vi "SMain.vi"() -> ()   [LabVIEW 2011] (continued)
      n242 = call "deleteFolder_vna.vi"("input_path"=w507) -> ()  [unwired: 1 in]
      n243 = Build Path(base path=w495, name or relative path="DelayConfig.txt" ("名称或相对路径")) -> (appended path=w493:path)
      n244 = call <vilib>:"Check if File or Folder Exists.vi"("path"=w493) -> ("file or folder exists?"=w492:bool, "dup path"=w491:path)  [unwired: 8 in, 1 out]
      n245 = call <vilib>:"Application Directory.vi"() -> ("Application Directory"=w516:path)
      n246 = constructor class="CPLTSApplicationClass"() -> (reference out=w504:refnum<k24>)  [unwired: 3 in, 2 out]
      n247 = call "equipconfirm.vi"("path to XML document"=w458) -> ("确认结果"=w457:bool)
      n248 = Build Path(base path=w516, name or relative path="Database\\LabelList.xlsx" ("名称或相对路径")) -> (appended path=w514:path)
      n249 = call <vilib>:"Check if File or Folder Exists.vi"("path"=w514) -> ("error out"=w511:errorcluster, "file or folder exists?"=w513:bool, "dup path"=w512:path)  [unwired: 8 in]
      n250 = local read "打印模式"() -> (w503:enum16{"IT Print", "EE Print"})
      n251 = case shown="假" w457 {
        frame False {
          n252 = Quit LabVIEW(quit? (T)=TRUE ("退出？(T)")) -> ()
        }
        frame True {
        }
      }
      n253 = control-ref of="Test Status:"() -> (w414:refnum<vi>)
      n254 = case shown="真" w492 {
        tunnel: w491 -> [w553 w564]
        frame False {
          w549 = 100.0 ("写入延时（单位：ms）")
          w550 = 100.0 ("读取延时（单位：ms）")
          n255 = local write "读取延时（单位：ms）"(w550) -> ()
          n256 = global write "延时设置全局变量.vi" "写入延时"(w550) -> ()
          n257 = local write "Q写入延时（单位：ms）"(250.0 ("写入延时（单位：ms）")) -> ()
          n258 = local write "S写入延时（单位：ms）"(w549) -> ()
          n259 = global write "延时设置全局变量.vi" "写入延时"(w549) -> ()
          n260 = call-poly <vilib>:"Write To Spreadsheet File.vi"("2D data"=string[][] [["Q写入延时时间（ms）：", "250"], ["S写入延时时间（ms）：", "100"], ["读取延时时间（ms）：", "100"]], "file path (dialog if empty)"=w553) -> ()  [unwired: 6 in, 1 out]
        }
        frame True {
          n261 = call-poly <vilib>:"Read From Spreadsheet File.vi"("file path (dialog if empty)"=w564) -> ("all rows"=w563:string[][])  [unwired: 6 in, 4 out]
          n262 = Index Array(array=w563, index (col)=1 ("禁用的索引 (列)")) -> (element=w561:string[])  [unwired: 1 in]
          n263 = Index Array(array=w561, index #1=0 ("索引")) -> (element #1=w559:string, element #2=w557:string, element #3=w556:string)  [unwired: 2 in]
          n264 = Fract/Exp String To Number(string=w559) -> (number=w554:dbl)  [unwired: 3 in, 1 out]
          n265 = Fract/Exp String To Number(string=w556) -> (number=w558:dbl)  [unwired: 3 in, 1 out]
          n266 = Fract/Exp String To Number(string=w557) -> (number=w555:dbl)  [unwired: 3 in, 1 out]
          n267 = local write "Q写入延时（单位：ms）"(w554) -> ()
          n268 = global write "延时设置全局变量.vi" "写入延时"(w554) -> ()
          n269 = local write "S写入延时（单位：ms）"(w555) -> ()
          n270 = local write "读取延时（单位：ms）"(w558) -> ()
          n271 = global write "延时设置全局变量.vi" "读取延时"(w558) -> ()
        }
      }
      n272 = invoke class="CPLTSApplicationClass" method="ShowWindow"(reference=w504, "nCmdShow"="nCmdShow") -> (reference out=w506:refnum<k24>)  [unwired: 2 in, 3 out]
      n273 = case shown="\"IT Print\", 默认" w503 {
        frame "IT Print", Default {
          n274 = property on="MO:" class="Str"("Visible"=TRUE ("可见")) -> ()  [unwired: 2 in, 2 out]
        }
        frame "EE Print" {
          n275 = property on="MO:" class="Str"("Visible"=FALSE ("可见")) -> ()  [unwired: 2 in, 2 out]
        }
      }
      n276 = property on="属性节点" class="Str"(reference=w414, "Text.BGColor"=u32 16711680, "Text.TextColor"=u32 16448250) -> ()  [unwired: 1 in, 2 out]
      n277 = case shown="真" w482 {
        tunnel: w458 -> [_ w526]
        tunnel: [string[] ["net use \\\\172.200.20.86 Luxshare-ict /user:C040345", "\\\\172.20.20.86\\HuaweiData\\DataRoot\\XML", "net use \\\\172.20.20.113 mesuser /user:mesuser", "\\\\172.20.20.113\\emc\\HPTS\\VNA", "\\\\172.20.20.113\\emc\\HPTS\\SI", "false"] ("OutParaArray") w535] -> w481
        tunnel: [string[] ["false"] ("OutParaArray") w533] -> w464
        tunnel: ["A" ("node text") w529] -> w459
        tunnel: [string[] [] ("OutParaArray") w527] -> w443
        frame False {
        }
        frame True {
          w539 = "Mo" ("名称")
          w541 = "PN" ("名称")
          n278 = call "xmlConfigRead.vi"("path to XML document"=w526, "XPath expression"="//OtherPara/*") -> ("OutParaArray"=w533:string[])  [unwired: 2 out]
          n279 = call "xmlConfigRead.vi"("path to XML document"=w526, "XPath expression"="//UploadPara/*") -> ("OutParaArray"=w535:string[])  [unwired: 2 out]
          n280 = call "xmlConfigRead.vi"("path to XML document"=w526, "XPath expression"="//LastPartNo/*") -> ("OutParaVariant"=w543:variant)  [unwired: 2 out]
          n281 = call "xmlConfigRead.vi"("path to XML document"=w526, "XPath expression"="//LineID/Line/@Name") -> ("OutParaArray"=w524:string[])  [unwired: 2 out]
          n282 = call "xmlConfigRead.vi"("path to XML document"=w526, "XPath expression"="//DBSet/ConnectInfo/@*") -> ("OutParaArray"=w527:string[])  [unwired: 2 out]
          n283 = call "xmlConfigRead.vi"("path to XML document"=w526, "XPath expression"="//SystemList/CurrentNO/@Name") -> ("OutParaArray"=w531:string[])  [unwired: 2 out]
          n284 = Get Variant Attribute(Variant=w543, name=w541) -> (duplicate Variant=w544:variant, value=w542:variant)  [unwired: 2 in, 2 out]
          n285 = Get Variant Attribute(Variant=w544, name=w539) -> (value=w540:variant)  [unwired: 2 in, 3 out]
          n286 = property on="线别" class="Ring (严格)"("Strings []"=w524) -> ()  [unwired: 2 in, 2 out]
          n287 = Variant To Data(type=w539, Variant=w540) -> (data=w537:string)  [unwired: 1 in, 1 out]
          n288 = Variant To Data(type=w541, Variant=w542) -> (data=w538:string)  [unwired: 1 in, 1 out]
          n289 = property on="P/N:" class="Str"("Val(Sgnl)"=w538) -> ()  [unwired: 2 in, 2 out]
          n290 = local write "MO:"(w537) -> ()
          n291 = Index Array(array=w531, index=0 ("索引")) -> (element=w529:string)
        }
      }
      "SystemMode" <- w459
      n292 = case shown="假" w513 {
        tunnel: w512 -> [w576 _]
        tunnel: w511 -> [_ _]
        frame False {
          n293 = call <vilib>:"New Report.vi"("report type"=T16."Excel") -> ("report out"=w578:refnum<class "NI_report.lvclass">)  [unwired: 13 in, 1 out]
          n294 = call <vilib>:"Excel Get Worksheet.vi"("report in"=w578, "worksheet index (0)"=0) -> ("report out"=w580:refnum<class "NI_report.lvclass">, "error out"=w579:errorcluster)  [unwired: 12 in]
          n295 = Build Array(string[] ["料号", "日期类型", "年份起始位", "年份结束位", "周起始位", "周结束位", "月份起始位", "月份结束位", "天数起始位", "天数结束位", "流水号起始位", "流水号起始位"]) -> (w573:string[][])
          n296 = call-poly <vilib>:"Excel Easy Table.vi"("report in"=w580, "text data"=w573, "error in (no error)"=w579) -> ("report out"=w575:refnum<class "NI_report.lvclass">)  [unwired: 8 in, 4 out]
          n297 = call-dynamic "Save Report to File.vi"("report in"=w575, "report file path"=w576) -> ("report out"=w583:refnum<class "NI_report.lvclass">, "error out"=w582:errorcluster)  [unwired: 12 in]
          n298 = call-dynamic "Dispose Report.vi"("report in"=w583, "wait until printing completed? (T)"=TRUE, "error in (no error)"=w582) -> ()  [unwired: 12 in, 1 out]
        }
        frame True {
        }
      }
      n299 = local write "Excel?"(TRUE ("Excel?")) -> ()
      n300 = local write "upload"(TRUE ("upload")) -> ()
      n301 = invoke class="CPLTSApplicationClass" method="CloseAllFiles"(reference=w506) -> ()  [unwired: 2 in, 3 out]
      n302 = constructor class="LabelPrintHelper"() -> (reference out=→"PRINT":refnum<k24>)  [unwired: 3 in, 2 out]
      n303 = constructor class="MESDataServices"() -> (reference out=→"SN":refnum<k24>)  [unwired: 3 in, 2 out]
      n304 = Delete From Array(array=w443, length=4 ("长度")) -> (deleted portion=w434:string[], array with subset deleted=w442:string[])  [unwired: 1 in]
      n305 = Index Array(array=w442) -> (element #1=w441:string, element #2=w440:string, element #3=w438:string, element #4=w439:string)  [unwired: 4 in]
      n306 = global write "全局.vi" "print templete"(FALSE ("print templete")) -> ()
      n307 = call "DES.vi"("sourceData"=w438, "操作"=enum16{"DES_Encrypt", "DES_Decrypt"}."DES_Decrypt") -> ("加密后字符串"=w437:string)  [unwired: 8 in, 1 out]
      n308 = Index Array(array=w464, index #1=0 ("索引"), index #2=1 ("索引"), index #3=2 ("索引"), index #4=3 ("索引")) -> (element #1=w461:string, element #2=w454:string, element #3=w450:string, element #4=w445:string)
      n309 = Decimal String To Number(string=w445) -> (number=→"startSN":i32)  [unwired: 2 in, 1 out]
      n310 = Bundle By Name(cluster=w433, "Server"=w441, "DB"=w440, "PSW"=w437, "User"=w439) -> (→"DB1":T8)
      n311 = Decimal String To Number(string=w454) -> (number=w453:i32)  [unwired: 2 in, 1 out]
      n312 = Equal?(x=w461, y="true") -> (x = y?=→"ConvertStyle":bool)
      n313 = Index Array(array=w481, index #1=0 ("索引"), index #2=1 ("索引"), index #3=2 ("索引"), index #4=3 ("索引"), index #5=4 ("索引"), index #6=5 ("索引"), index #7=6 ("索引"), index #8=7 ("索引"), index #9=8 ("索引")) -> (element #1=→"NetCmd":string, element #2=→"NetPathHW":string, element #3=→"NetCmdCompress":string, element #4=w473:string, element #5=w472:string, element #6=w468:string, element #7=w420:string, element #8=→"NetTemppath":string, element #9=→"NetLocalpath":string)
      n314 = String To Path(string=w473) -> (path=→"NetPathCompress1":path)
      n315 = String To Path(string=w472) -> (path=→"NetPathCompress2":path)
      n316 = Equal?(x=w450, y="true") -> (x = y?=→"TestResultSave":bool)
      n317 = global write "全局.vi" "logsetting"(w453) -> ()
      n318 = Equal?(x=w468, y="true") -> (x = y?=→"AlarmDisplay":bool)
      n319 = Index Array(array=w434) -> (element #1=w432:string, element #2=w431:string, element #3=w429:string, element #4=w427:string)  [unwired: 4 in]
      n320 = call "DES.vi"("sourceData"=w429, "操作"=enum16{"DES_Encrypt", "DES_Decrypt"}."DES_Decrypt") -> ("加密后字符串"=w430:string)  [unwired: 8 in, 1 out]
      n321 = Equal?(x=w420, y="true") -> (x = y?=→"asychronus":bool)
      n322 = Bundle By Name(cluster=w433, "Server"=w432, "DB"=w431, "PSW"=w430, "User"=w427) -> (→"DB2":T8)
    }
    frame #5 {
      n323 = property on="Type" class="Ring (严格)"("Val(Sgnl)"=u16 0 ("值(信号)")) -> ()  [unwired: 2 in, 2 out]
      n324 = property on="Start Test" class="Bool"("BoolText.Text"="START TEST" ("布尔文本.文本")) -> ()  [unwired: 2 in, 2 out]
      n325 = local write "caliDataSelect"(FALSE ("caliDataSelect")) -> ()
    }
    frame #6 {
      n326 = while {
        tunnel: [w590] -> _
        stop <- w590 stop-if-true
        n327 = case shown="\"test\"" "State" {
          tunnel: [_ _ TRUE ("Stop") w1944] -> w590
          frame "test" {
            n328 = stacked-sequence {
              frame #0 {
                n329 = property on="Start Test" class="Bool"("DisabledEnum"=2) -> ()  [unwired: 2 in, 2 out]
                n330 = local write "proBar"(u8 0 ("proBar")) -> ()
                n331 = local write "preStation"("" ("preStation")) -> ()
                n332 = property on="preStation" class="Str"("Visible"=FALSE ("可见")) -> ()  [unwired: 2 in, 2 out]
                n333 = control-ref of="Test Status:"() -> (w592:refnum<vi>)
                n334 = property on="属性节点" class="Str"(reference=w592, "Text.BGColor"=u32 16448250, "Text.TextColor"=u32 0) -> ()  [unwired: 1 in, 2 out]
                n335 = property on="S/N:" class="Str"("DisabledEnum"=T17."Disabled and Grayed Out" ("禁用")) -> ()  [unwired: 2 in, 2 out]
                n336 = local write "strFSN 原始SN"("" ("strFSN 原始SN")) -> ()
                n337 = local write "Current Testing Label/当前测试条码"("") -> ()
                n338 = local write "midVar_time_date"(timestamp(3534465477 s since 1904-01-01) ("midVar_time_date")) -> ()
                n339 = local write "未经进制转换的sn(客户 jin zhi sn)"("" ("未经进制转换的sn(客户 jin zhi sn)")) -> ()
                n340 = local write "Test Status:"("" ("Test Status:")) -> ()
                n341 = local write "要烧录的DateCode"("" ("要烧录的DateCode")) -> ()
                n342 = local write "要烧录的时间和Sn"("" ("要烧录的时间和Sn")) -> ()
                "customer date" <- "" ("customer date")
                "Shi jin zhi sn" <- "" ("Shi jin zhi sn")
              }
              frame #1 {
                n343 = local read "Use Counts?"() -> (w610:bool)
                n344 = case shown="真" w610 {
                  tunnel: [TRUE w613] -> w609
                  frame False {
                  }
                  frame True {
                    n345 = stacked-sequence {
                      seq-local: [w616 _] -> [_ w624]
                      seq-local: [w615 _] -> [_ w621]
                      tunnel: [_ w620] -> w613
                      frame #0 {
                        n346 = local read "RS232 I2C Counts"() -> (w614:refnum<visa-resource-name>)
                        n347 = call "读取使用次数和寿命.vi"("截取长度"=4, "开始截取位"=8, "VISA  2"=w614) -> ("result"=w616:bool, "Data Out"=w615:u8[], "无符号字节数组"=→"无符号字节数组":u8[])  [unwired: 6 in]
                        "Data Out  2" <- w615
                        "result" <- w616
                      }
                      frame #1 {
                        # "读取使用次数错误吗？"
                        n348 = Equal?(x=FALSE, y=w624) -> (x = y?=w622:bool)
                        n349 = case shown="假" w622 {
                          tunnel: w621 -> [w643 _]
                          tunnel: [w636 FALSE] -> w620
                          frame False {
                            w630 = 256
                            # "使用次数大于寿命"
                            n350 = Index Array(array=w643, index #1=0 ("索引"), index #2=1 ("索引"), index #3=2 ("索引"), index #4=3 ("索引")) -> (element #1=w635:u8, element #2=w639:u8, element #3=w633:u8, element #4=w638:u8)
                            n351 = Multiply(x=w630, y=w635) -> (x*y=w634:i32)
                            n352 = Multiply(x=w630, y=w633) -> (x*y=w632:i32)
                            n353 = Add(x=w632, y=w638) -> (x+y=w629:i32)
                            n354 = Add(x=w634, y=w639) -> (x+y=w628:i32)
                            n355 = Subtract(x=w629, y=w628) -> (x-y=w627:i32)
                            n356 = Less?(x=w627, y=200) -> (x < y?=w625:bool)
                            n357 = case shown="真" w625 {
                              frame False {
                              }
                              frame True {
                                n358 = One Button Dialog(message="计数板可使用次数小于200,请注意！" ("消息")) -> ()  [unwired: 1 in, 1 out]
                              }
                            }
                            n359 = Greater?(x=w628, y=w629) -> (0:w637:bool)
                            n360 = case shown="假" w637 {
                              tunnel: [w646 FALSE] -> w636
                              frame False {
                                n361 = local read "RS232 I2C Counts"() -> (w645:refnum<visa-resource-name>)
                                n362 = call "使用次数加1.vi"("VISA  2"=w645) -> ("result"=w646:bool)  [unwired: 10 in]
                              }
                              frame True {
                              }
                            }
                            n363 = local write "UseAge"(w629) -> ()
                            n364 = local write "Used"(w628) -> ()
                          }
                          frame True {
                            n365 = One Button Dialog(message="测试板使用次数读取错误！") -> ()  [unwired: 1 in, 1 out]
                          }
                        }
                      }
                    }
                  }
                }
                n366 = local write "test time"(string[] [] ("test time")) -> ()
                n367 = case shown="真" w609 {
                  frame False {
                    # "测试版使用次数是否合格"
                    n368 = local read "UseAge"() -> (w654:i64)
                    n369 = local read "Used"() -> (w657:i64)
                    n370 = local write "Go"(FALSE ("Go")) -> ()
                    n371 = Number To Decimal String(number=w657) -> (decimal integer string=w656:string)  [unwired: 1 in]
                    n372 = Number To Decimal String(number=w654) -> (decimal integer string=w653:string)  [unwired: 1 in]
                    n373 = Concatenate Strings("测试板使用了", w656, "次,超过了最大使用寿命:" ("字符串"), w653, "不允许继续使用，请更换测试板后继续测试！" ("字符串"), "或者修改使用次数的动作失败！" ("字符串")) -> (w651:string)
                    n374 = One Button Dialog(message=w651) -> ()  [unwired: 1 in, 1 out]
                  }
                  frame True {
                    # "测试版使用次数是否合格"
                    n375 = local read "线别确认"() -> (w661:bool)
                    n376 = Not(x=w661) -> (.not. x?=w660:bool)
                    n377 = case shown="假" w660 {
                      frame False {
                        n378 = control-ref of="Test Status:"() -> (w667:refnum<vi>)
                        n379 = property class="Str"(reference=w667) -> (reference out=w665:refnum<vi>, "Value"=w668:string)  [unwired: 1 in, 1 out]
                        n380 = local read "DateCode8Value_0X30"() -> (w662:i32)
                        n381 = local read "打印模式"() -> (w671:enum16{"IT Print", "EE Print"})
                        n382 = local read "AutoSN"() -> (w672:bool)
                        n383 = local read "ConvertStyle"() -> (w670:bool)
                        n384 = Number To Hexadecimal String(2:w662) -> (0:w663:string)  [unwired: 1 in]
                        n385 = Concatenate Strings(w668, "\n", "当前datacode为:0X", w663) -> (w666:string)
                        n386 = property class="Str"(reference=w665, "Value"=w666) -> ()  [unwired: 1 in, 2 out]
                        n387 = case shown="假" w672 {
                          tunnel: w671 -> [_ w729]
                          tunnel: w670 -> [w682 w728]
                          tunnel: w662 -> [w681 w727]
                          frame False {
                            # "前站数据是否需要管控"
                            n388 = local read "S/N:"() -> (w679:string)
                            n389 = local read "P/N:"() -> (w674:string)
                            n390 = local read "DB1"() -> (w678:T8)
                            n391 = call "前站查询(T1).vi"("Station"="preStation", "Pre Check"="Pre Check", "PN"=w674, "DBSet"=w678, "SN"=w679) -> ("判定"=w677:bool)  [unwired: 6 in]
                            n392 = call "前站查询.vi"("DBSet"=w678, "SN"=w679) -> ("判定"=w676:bool)  [unwired: 9 in]
                            n393 = And(x=w676, y=w677) -> (x .and. y?=w675:bool)
                            n394 = case shown="真" w675 {
                              tunnel: w682 -> [_ w686]
                              tunnel: w681 -> [_ w685]
                              frame False {
                                n395 = One Button Dialog(message="前面有不良维修记录待处理，请进行处理后再测试" ("消息")) -> ()  [unwired: 1 in, 1 out]
                                n396 = local write "Go"(FALSE ("Go")) -> ()
                              }
                              frame True {
                                n397 = stacked-sequence {
                                tunnel: w686 -> [_ w694]
                                tunnel: w685 -> [_ w693]
                                frame #0 {
                                n398 = local read "DB1"() -> (w687:T8)
                                n399 = local read "LastSN"() -> (w691:string)
                                n400 = local read "S/N:"() -> (w690:string)
                                n401 = call "重测.vi"("Last SN"=w691, "DBSet"=w687, "SN"=w690) -> ("继续?"=→"继续?":bool, "重测原因"=→"重测原因":string)  [unwired: 6 in, 1 out]
                                }
                                frame #1 {
                                n402 = local read "继续?"() -> (w692:bool)
                                n403 = case shown="真" w692 {
                                tunnel: w694 -> [_ w706]
                                tunnel: w693 -> [_ w705]
                                frame False {
                                n404 = local write "Go"(FALSE ("Go")) -> ()
                                }
                                frame True {
                                # "20160919增加从labelprint表查询，理由：作业流程变更，第一站就打条码。"
                                # "针对重工已经打印标签\n的进行修改，从资讯\n数据库中查到SN对应\n的信息回来进行测试"
                                n405 = local read "DB1"() -> (w703:T8)
                                n406 = local read "P/N:"() -> (w725:string)
                                n407 = local read "Local Database"() -> (w697:bool)
                                n408 = local read "mid_str_labelType"() -> (w723:string)
                                n409 = local read "labelConfig"() -> (w722:string[])
                                n410 = local read "打印模式"() -> (w700:enum16{"IT Print", "EE Print"})
                                n411 = local read "校验信息"() -> (w702:T7)
                                n412 = Equal?(x=w700, y=enum16{"IT Print", "EE Print"}."EE Print") -> (x = y?=w698:bool)
                                n413 = Or(x=w697, y=w698) -> (x .or. y?=w696:bool)
                                n414 = local read "S/N:"() -> (w724:string)
                                "LastSN" <- w724
                                n415 = local read "mid_array_eep"() -> (w721:string[][])
                                n416 = call "精简框图4.vi"("P/N:"=w725, "mid_str_labelType"=w723, "DateCode8Value_0X30"=w705, "Convert Style"=w706, "LocalDataBase?"=w696, "labelConfig"=w722, "mid_array_eep"=w721, "SNKeep"="SN Keep", "S/N"=w724, "DBSet"=w703, "校验信息"=w702) -> ("show_date"=w710:timestamp, "要烧录的时间和Sn"=w720:string, "未经进制转换的sn(客户 jin zhi sn)"=w711:string, "要烧录的DateCode"=w719:string, "strFSN 原始 Customer sn"=w712:string, "输出的label内容"=w709:string, "Go"=w708:bool, "mid_array_temp_int"=w718:u8[][], "S/N:"=w717:string, "Customer Date"=w716:string, "shi jin zhi sn"=w715:string, "Report No."=w714:string, "Sample #"=w713:string)  [unwired: 4 in]
                                n417 = And(x=w708, y=TRUE) -> (x .and. y?=w707:bool)
                                n418 = local write "Go"(w707) -> ()
                                n419 = local write "midVar_time_date"(w710) -> ()
                                n420 = local write "strFSN 原始SN"(w712) -> ()
                                n421 = local write "未经进制转换的sn(客户 jin zhi sn)"(w711) -> ()
                                n422 = local write "要烧录的时间和Sn"(w720) -> ()
                                n423 = local write "要烧录的DateCode"(w719) -> ()
                                n424 = local write "Current Testing Label/当前测试条码"(w709) -> ()
                                n425 = local write "mid_array_temp_int"(w718) -> ()
                                n426 = local write "S/N:"(w717) -> ()
                                n427 = local write "customer date"(w716) -> ()
                                n428 = local write "Shi jin zhi sn"(w715) -> ()
                                n429 = local write "Report No."(w714) -> ()
                                n430 = local write "Sample #"(w713) -> ()
                                n431 = local write "midVar_str_SN"(w709) -> ()
                                }
                                }
                                }
                                }
                              }
                            }
                          }
                          frame True {
                            n432 = local write "重测原因"("firsttest" ("重测原因")) -> ()
                            n433 = case shown="\"IT Print\", 默认" w729 {
                              tunnel: w728 -> [w733 w762]
                              tunnel: w727 -> [w731 w756]
                              frame "IT Print", Default {
                                # "没有转进制的流水"
                                # "mid_array_temp_int 是展开后的烧录文件"
                                # "通过MIS获得Sn"
                                n434 = local read "MO:"() -> (w742:string)
                                n435 = local read "mid_str_labelType"() -> (w750:string)
                                n436 = local read "SN"() -> (w732:refnum<k24>)
                                n437 = local read "labelConfig"() -> (w749:string[])
                                n438 = local read "mid_array_eep"() -> (w748:string[][])
                                n439 = local read "P/N:"() -> (w751:string)
                                n440 = local read "校验信息"() -> (w730:T7)
                                n441 = call "精简框图3.vi"("P/N:"=w751, "mid_str_labelType"=w750, "DateCode8Value_0X30"=w731, "Convert Style"=w733, "新引用"=w732, "labelConfig"=w749, "mid_array_eep"=w748, "工单号"=w742, "校验信息"=w730) -> ("show_date"=w741:timestamp, "要烧录的时间和Sn"=→"要烧录的时间和Sn":string, "未经进制转换的sn(客户 jin zhi sn)"=w734:string, "要烧录的DateCode"=→"要烧录的DateCode":string, "strFSN 原始 Customer sn"=w737:string, "输出的label内容"=w740:string, "Go"=w743:bool, "mid_array_temp_int"=w747:u8[][], "S/N:"=w746:string, "Customer Date"=w736:string, "shi jin zhi sn"=w735:string, "Report No."=w745:string, "Sample #"=w744:string)  [unwired: 6 in]
                                "Current Testing Label/当前测试条码" <- w740
                                n442 = local write "mid_array_temp_int"(w747) -> ()
                                n443 = local write "S/N:"(w746) -> ()
                                n444 = local write "Report No."(w745) -> ()
                                n445 = local write "Sample #"(w744) -> ()
                                n446 = local write "midVar_str_SN"(w740) -> ()
                                n447 = local write "Go"(w743) -> ()
                                n448 = local write "midVar_time_date"(w741) -> ()
                                n449 = local write "未经进制转换的sn(客户 jin zhi sn)"(w734) -> ()
                                n450 = local write "strFSN 原始SN"(w737) -> ()
                                n451 = local write "customer date"(w736) -> ()
                                n452 = local write "Shi jin zhi sn"(w735) -> ()
                              }
                              frame "EE Print" {
                                n453 = local read "startSN"() -> (w753:i32)
                                n454 = control-ref of="Test Status:"() -> (w760:refnum<vi>)
                                n455 = local read "mid_str_labelType"() -> (w766:string)
                                n456 = local read "mid_str_snformat"() -> (w765:string)
                                n457 = local read "P/N:"() -> (w763:string)
                                n458 = local read "mid_array_eep"() -> (w761:string[][])
                                n459 = local read "校验信息"() -> (w752:T7)
                                n460 = property class="Str"(reference=w760) -> (reference out=w758:refnum<vi>, "Value"=w759:string)  [unwired: 1 in, 1 out]
                                n461 = call "精简框图1.vi"("mid_str_labelType"=w766, "mid_array_eep"=w761, "mid_str_snformat"=w765, "Convert Style"=w762, "DateCode8Value_0X30"=w756, "P/N"=w763, "Sart SN"=w753, "校验信息"=w752) -> ("LocalSN Generate Status"=w755:string, "midVar_time_date"=w767:timestamp, "midVar_str_SN"=w768:string, "mid_array_temp_int"=w769:u8[][], "S/N:"=w770:string, "Report No."=w771:string, "Sample #"=w772:string)  [unwired: 5 in]
                                n462 = Concatenate Strings(w759, "\n", w755) -> (w757:string)
                                n463 = local write "Go"(TRUE ("Go")) -> ()
                                n464 = local write "midVar_time_date"(w767) -> ()
                                n465 = local write "midVar_str_SN"(w768) -> ()
                                n466 = local write "mid_array_temp_int"(w769) -> ()
                                n467 = local write "S/N:"(w770) -> ()
                                n468 = local write "Report No."(w771) -> ()
                                n469 = local write "Sample #"(w772) -> ()
                                n470 = property class="Str"(reference=w758, "Value"=w757) -> ()  [unwired: 1 in, 2 out]
                              }
                            }
                          }
                        }
                      }
                      frame True {
                        n471 = disable-structure shown="禁用" {
                          frame Disabled {
                            # "前站数据是否需要管控"
                            n472 = local read "S/N:"() -> (w777:string)
                            n473 = call "subVI3_MAIN_checkBeforeTest_wmg.vi"("input_str_SN"=w777) -> ("show_bool_checkResult"=w776:bool, "show_str_failTable"=w778:string, "show_messageOut"=w775:string)  [unwired: 1 out]
                            n474 = case shown="真" w776 {
                              tunnel: w778 -> [w783 _]
                              tunnel: w775 -> [_ w788]
                              frame False {
                                w782 = "\n"
                                n475 = local write "Go"(FALSE ("Go")) -> ()
                                n476 = Concatenate Strings("工站", w782, w783, w782, "没有测试或者测试失败！") -> (w780:string)
                                n477 = One Button Dialog(message=w780) -> ()  [unwired: 1 in, 1 out]
                                n478 = local write "Test Status:"(w780) -> ()
                              }
                              frame True {
                                # "前站数据的查询结果"
                                n479 = local write "preStation"(w788) -> ()
                                n480 = local read "AutoSN"() -> (w786:bool)
                                n481 = property on="preStation" class="Str"("Visible"=TRUE ("可见")) -> ()  [unwired: 2 in, 2 out]
                                n482 = case shown="假" w786 {
                                frame False {
                                n483 = local read "mid_str_labelType"() -> (w792:string)
                                n484 = local read "mid_str_snformat"() -> (w791:string)
                                n485 = local read "mid_array_eep"() -> (w793:string[][])
                                n486 = local read "S/N:"() -> (w789:string)
                                n487 = local read "P/N:"() -> (w790:string)
                                n488 = call "精简框图2.vi"("S/N:"=w789, "P/N:"=w790, "mid_str_snformat"=w791, "mid_str_labelType"=w792, "mid_array_eep"=w793) -> ("Report No."=w794:string, "Sample #"=w795:string, "midVar_time_date"=w796:timestamp, "midVar_str_SN"=w797:string, "mid_array_temp_int"=w798:u8[][])  [unwired: 6 in]
                                n489 = local write "Report No."(w794) -> ()
                                n490 = local write "Sample #"(w795) -> ()
                                n491 = local write "midVar_time_date"(w796) -> ()
                                n492 = local write "midVar_str_SN"(w797) -> ()
                                n493 = local write "mid_array_temp_int"(w798) -> ()
                                }
                                frame True {
                                # "自动EE获取sn"
                                n494 = local read "mid_str_labelType"() -> (w801:string)
                                n495 = local read "mid_str_snformat"() -> (w800:string)
                                n496 = local read "mid_array_eep"() -> (w799:string[][])
                                n497 = call "精简框图1.vi"("mid_str_labelType"=w801, "mid_array_eep"=w799, "mid_str_snformat"=w800) -> ("midVar_time_date"=w802:timestamp, "midVar_str_SN"=w803:string, "mid_array_temp_int"=w804:u8[][], "S/N:"=w805:string, "Report No."=w806:string, "Sample #"=w807:string)  [unwired: 10 in, 1 out]
                                n498 = local write "midVar_time_date"(w802) -> ()
                                n499 = local write "midVar_str_SN"(w803) -> ()
                                n500 = local write "mid_array_temp_int"(w804) -> ()
                                n501 = local write "S/N:"(w805) -> ()
                                n502 = local write "Report No."(w806) -> ()
                                n503 = local write "Sample #"(w807) -> ()
                                }
                                }
                                n504 = local write "Go"(TRUE ("Go")) -> ()
                              }
                            }
                          }
                          frame Enabled {
                          }
                        }
                        n505 = local write "Go"(FALSE ("Go")) -> ()
                        n506 = One Button Dialog(message="线别未确认" ("消息")) -> ()  [unwired: 1 in, 1 out]
                      }
                    }
                  }
                }
              }
              frame #2 {
                n507 = local read "Go"() -> (w808:bool)
                n508 = case shown="真" w808 {
                  frame False {
                    w812 = 0
                    n509 = property on="S/N:" class="Str"("Key Focus"=TRUE ("键选中")) -> ()  [unwired: 2 in, 2 out]
                    n510 = local write "State"("wait" ("state")) -> ()
                    n511 = local write "S/N:"("") -> ()
                    n512 = property on="S/N:" class="Str"("DisabledEnum"=T17."Enabled" ("禁用")) -> ()  [unwired: 2 in, 2 out]
                    n513 = property on="Start Test" class="Bool"("DisabledEnum"=w812) -> ()  [unwired: 2 in, 2 out]
                    n514 = property on="Tab_Graph" class="TabCtl (严格)"("Value"=w812) -> ()  [unwired: 2 in, 2 out]
                  }
                  frame True {
                    n515 = local read "P/N:"() -> (w818:string)
                    n516 = local read "VNA Model:"() -> (w824:enum16{"E5071C", "N5230A(C)", "N5224A"})
                    n517 = local read "Spec _Col"() -> (w819:i32[])
                    n518 = control-ref of="Test Status:"() -> (w823:refnum<vi>)
                    n519 = local read "VNA VISA"() -> (w825:refnum<visa-resource-name>)
                    n520 = local read "S/N:"() -> (w822:string)
                    n521 = call "Sample name judge.vi"("Sample  Name:"=w818, "START input"=TRUE) -> ("START output"=w826:bool)
                    n522 = case shown="真" w826 {
                      tunnel: "DAQ Device" -> [_ w846]
                      tunnel: w825 -> [_ w845]
                      tunnel: w824 -> [_ w844]
                      tunnel: w823 -> [_ w843]
                      tunnel: w822 -> [_ w842]
                      tunnel: "Port Type" -> [_ w841]
                      tunnel: "Demo" -> [_ w840]
                      tunnel: w819 -> [_ w839]
                      tunnel: w818 -> [_ w838]
                      tunnel: "Manual" -> [_ w837]
                      tunnel: "VISA COM" -> [_ w836]
                      tunnel: "DAQ  Model:" -> [_ w835]
                      tunnel: "Crosstalk  by Trace" -> [_ w834]
                      frame False {
                        w833 = 0
                        n523 = property on="S/N:" class="Str"("Key Focus"=TRUE ("键选中")) -> ()  [unwired: 2 in, 2 out]
                        n524 = local write "State"("wait" ("state")) -> ()
                        n525 = local write "S/N:"("") -> ()
                        n526 = property on="Start Test" class="Bool"("DisabledEnum"=w833) -> ()  [unwired: 2 in, 2 out]
                        n527 = property on="S/N:" class="Str"("DisabledEnum"=T17."Enabled" ("禁用")) -> ()  [unwired: 2 in, 2 out]
                        n528 = property on="Tab_Graph" class="TabCtl (严格)"("Value"=w833) -> ()  [unwired: 2 in, 2 out]
                      }
                      frame True {
                        n529 = stacked-sequence {
                          seq-local: [_ _ _ _ _ _ _ _ _ _ w1501 _ _ _ _ _ _] -> [_ _ _ _ _ _ _ _ _ _ _ w1526 _ _ _ _ _]
                          tunnel: w846 -> [_ _ _ w987 w1128 w1223 _ _ _ _ _ w1545 _ _ _ _ _]
                          tunnel: w845 -> [_ _ _ w986 w1127 w1222 _ _ _ _ _ _ _ _ _ _ _]
                          tunnel: w844 -> [_ _ _ w985 w1126 w1221 _ _ _ _ _ _ _ _ _ _ _]
                          tunnel: w838 -> [_ _ w930 w984 w1125 w1220 _ _ _ _ _ _ _ _ _ _ _]
                          tunnel: w843 -> [_ _ w911 w983 w1124 w1219 _ _ w1343 w1407 w1503 w1543 w1593 _ w1789 _ _]
                          tunnel: w842 -> [_ _ w922 w982 w1123 w1218 _ _ _ _ _ _ _ _ _ _ _]
                          tunnel: w841 -> [_ _ _ w976 w1121 w1216 _ _ _ _ _ _ _ _ _ _ _]
                          tunnel: w840 -> [_ _ _ w966 w1111 w1206 _ w1323 _ w1405 _ w1538 _ _ w1784 w1840 _]
                          tunnel: w839 -> [_ _ _ w975 w1122 w1217 _ _ _ _ _ _ _ _ _ _ _]
                          tunnel: w837 -> [_ _ _ w965 w1110 w1205 _ _ _ _ _ w1539 _ _ _ _ _]
                          tunnel: w836 -> [_ _ _ w971 w1117 w1211 _ _ _ _ _ w1536 _ _ _ _ _]
                          tunnel: w835 -> [_ _ _ w970 w1116 w1210 _ _ _ _ _ w1535 _ _ _ _ _]
                          tunnel: w834 -> [_ _ w908 _ w1114 w1209 _ _ _ _ _ _ _ _ _ _ _]
                          frame #0 {
                            n530 = call <vilib>:"Application Directory.vi"() -> ("Application Directory"=w862:path)
                            n531 = Build Path(base path=w862, name or relative path="Database\\yellowLabelPN.txt" ("名称或相对路径")) -> (appended path=w860:path)
                            n532 = call <vilib>:"Check if File or Folder Exists.vi"("path"=w860) -> ("error out"=w857:errorcluster, "file or folder exists?"=w859:bool, "dup path"=w858:path)  [unwired: 8 in]
                            n533 = case shown="假" w859 {
                              tunnel: w858 -> [w869 w875]
                              tunnel: [w868 w876] -> _
                              tunnel: w857 -> [w867 w876]
                              tunnel: [w866 w875] -> w850
                              frame False {
                                n534 = stacked-sequence {
                                tunnel: w869 -> [w873 w874]
                                tunnel: [w872 _] -> w868
                                tunnel: w867 -> [w871 _]
                                tunnel: [_ w874] -> w866
                                frame #0 {
                                n535 = Write to Text File(file (use dialog)=w873, text="LR44" ("文本"), error in=w871) -> (error out=w872:errorcluster)  [unwired: 1 in, 2 out]
                                }
                                frame #1 {
                                }
                                }
                              }
                              frame True {
                              }
                            }
                            n536 = call-poly <vilib>:"Read From Spreadsheet File.vi"("file path (dialog if empty)"=w850) -> ("all rows"=w856:string[][])  [unwired: 6 in, 4 out]
                            n537 = Index Array(array=w856, index (col) #1=0 ("禁用的索引 (列)"), index (col) #2=1 ("索引 (列)")) -> (element #1=w854:string[], element #2=w848:string[])  [unwired: 2 in]
                            n538 = local read "P/N:"() -> (w853:string)
                            n539 = Search 1D Array(1D array=w854, element=w853) -> (index of element=w847:i32)  [unwired: 1 in]
                            n540 = Not Equal?(x=w847, y=-1) -> (x != y?=w851:bool)
                            n541 = case shown="真" w851 {
                              tunnel: w848 -> [_ w865]
                              tunnel: w847 -> [_ w864]
                              frame False {
                              }
                              frame True {
                                n542 = Index Array(array=w865, index=w864) -> (element=w863:string)
                                n543 = call "yellowLabelDialog.vi"("图片路径"=w863) -> ()  [unwired: 11 in]
                              }
                            }
                          }
                          frame #1 {
                            w881 = 8 ("y")
                            n544 = disable-structure shown="禁用" {
                              frame Disabled {
                                n545 = local read "Diff Test Item Name"() -> (w885:string[])
                                n546 = call "Divide Test Items.vi"("Test Item Name"=w885) -> ()  [unwired: 9 in, 2 out]
                              }
                              frame Enabled {
                              }
                            }
                            n547 = local read "S-Para Item List"() -> (w877:string[])
                            n548 = local write "db_ResultString"("") -> ()
                            n549 = Array Size(array=w877) -> (size(s)=w882:i32)
                            n550 = local read "Test Graph"() -> (w880:refnum<vi>[])
                            n551 = local read "Empty"() -> (w879:cluster{"Horz Time array":dbl[], "Y":dbl[]}[])
                            n552 = Less Or Equal?(x=w882, y=w881) -> (x <= y?=w883:bool)
                            n553 = Select(t=w882, s=w883, f=w881) -> (s? t:f=w884:i32)
                            n554 = for {
                              tunnel: w880 -> [w891] mode=indexing
                              tunnel: w879 -> [w890]
                              tunnel: w884 -> [w887]
                              tunnel: w877 -> [w889]
                              i -> [w886]
                              n555 = Index Array(array=w889, index=w886) -> (element=w888:string)
                              n556 = Less?(x=w886, y=w887) -> (x < y?=w892:bool)
                              n557 = case shown="假" w892 {
                                tunnel: w891 -> [w894 w898]
                                tunnel: w890 -> [w893 w897]
                                tunnel: w888 -> [_ w896]
                                frame False {
                                n558 = property class="XYGraph (严格)"(reference=w894, "Value"=w893, "Caption.Visible"=FALSE ("标题.可见")) -> ()  [unwired: 1 in, 2 out]
                                }
                                frame True {
                                n559 = property class="XYGraph (严格)"(reference=w898, "Value"=w897, "Caption.Visible"=TRUE ("标题.可见"), "Caption.Text"=w896) -> ()  [unwired: 1 in, 2 out]
                                }
                              }
                            }
                          }
                          frame #2 {
                            w903 = FALSE ("Urgent Stop")
                            w926 = 8 ("y")
                            n560 = stacked-sequence {
                              frame #0 {
                                n561 = local write "db_VNA"("" ("db_VNA")) -> ()
                              }
                              frame #1 {
                                w938 = ";" ("字符串")
                                n562 = local read "P/N:"() -> (w939:string)
                                n563 = local read "S/N:"() -> (w940:string)
                                n564 = Concatenate Strings(w939, w938, w940, w938) -> (w941:string)
                                n565 = local write "db_VNA"(w941) -> ()
                              }
                            }
                            n566 = local read "Dem 2X"() -> (w904:bool)
                            n567 = local read "S-Para Item List"() -> (w902:string[])
                            n568 = local read "2x equalize"() -> (w901:bool)
                            n569 = Bundle("Urgent Stop"=FALSE, "Crosstalk  by Trace"=w908, "Dem 2X"=w904, "2x equalize"=w901) -> (→"Option":T20)  [unwired: 1 in]
                            n570 = stacked-sequence {
                              tunnel: w911 -> [w956 w961]
                              tunnel: w930 -> [_ w960]
                              tunnel: w922 -> [_ w959]
                              frame #0 {
                                w957 = u16 1 items=["Normal Input", "Start", "Product Inf", "End"] ("Summary Method")
                                n571 = call "Summary Generating.vi"("Summary Method"=w957, "Status String"=w956) -> ()  [unwired: 26 in]
                              }
                              frame #1 {
                                w962 = u16 2 items=["Normal Input", "Start", "Product Inf", "End"] ("Summary Method")
                                n572 = local read "Length"() -> (w958:string)
                                n573 = call "Summary Generating.vi"("Summary Method"=w962, "Status String"=w961, "Sample S/N:"=w959, "Sample PN:"=w960, "Length(mm)"=w958) -> ()  [unwired: 23 in]
                              }
                            }
                            n574 = local read "Test Graph"() -> (w912:refnum<vi>[])
                            n575 = control-ref of="Tab_Graph"() -> (w913:refnum<vi>)
                            n576 = control-ref of="db_ResultString"() -> (w906:refnum<vi>)
                            n577 = Array Size(array=w902) -> (size(s)=w924:i32)
                            "S Item Size" <- w924
                            n578 = Get Date/Time In Seconds() -> (seconds since 1Jan1904=→"Start Time":timestamp)
                            n579 = Bundle("Tab_Graph"=w913, "Test Graph"=w912, "Test Status:"=w911, "db_ResultString"=w906) -> (→"Reference":T5)  [unwired: 1 in]
                            n580 = local write "Urgent Stop"(w903) -> ()
                            n581 = global write "全局.vi" "manual stop"(w903) -> ()
                            n582 = Get Date/Time In Seconds() -> (seconds since 1Jan1904=→"start":timestamp)
                            n583 = local read "TDR Test Item Name"() -> (w920:string[])
                            n584 = property on="Urgent Stop" class="Bool (严格)"("DisabledEnum"=0 ("索引")) -> ()  [unwired: 2 in, 2 out]
                            n585 = local read "S-para Pair Name"() -> (w936:string[])
                            n586 = property on="Start Test" class="Bool"("DisabledEnum"=2) -> ()  [unwired: 2 in, 2 out]
                            n587 = local read "NEXT Pair Name"() -> (w934:string[])
                            n588 = local read "FEXT Pair Name"() -> (w932:string[])
                            n589 = local read "Test Graph"() -> (w928:refnum<vi>[])
                            n590 = Array Size(array=w932) -> (size(s)=→"F-Pair Loop":i32)
                            n591 = Array Size(array=w934) -> (size(s)=→"N-Pair Loop":i32)
                            n592 = Array Size(array=w936) -> (size(s)=→"S-Pair Loop":i32)
                            n593 = Array Size(array=w920) -> (size(s)=→"T Item Size":i32)
                            n594 = Less Or Equal?(x=w924, y=w926) -> (x <= y?=w927:bool)
                            n595 = local read "Empty"() -> (w923:cluster{"Horz Time array":dbl[], "Y":dbl[]}[])
                            n596 = Select(t=w924, s=w927, f=w926) -> (s? t:f=w925:i32)
                            n597 = for {
                              tunnel: w928 -> [w947] mode=indexing
                              tunnel: w923 -> [w946]
                              tunnel: w925 -> [w943]
                              tunnel: w902 -> [w945]